vi "RX TX Open (N Channel).vi"(0 "resources":T15[](array[typedef]), 1 "option string":string, 3 "direction":T12, 9 "session in":T1[](array[typedef]), 11 "error in":errorcluster, 12 "force download":bool) -> (4 "tx baseband session out":T2[](array[typedef]), 6 "rx baseband session out":T10[](array[typedef]), 10 "session out":T1[](array[typedef]), 15 "error out":errorcluster)   [LabVIEW 2019]
uses:
  TypeDefs/Resources.ctl
  <vilib>/userDefined/High Color/nirio_resource_hc.ctl
  TypeDefs/Tx Baseband Session.ctl
  <instrlib>/niMmWave/ni3610 and ni3630/controls/public/Main Settings.ctl
  <vilib>/Instr/_visa.llb/VISA Register Access Address Space.ctl
  <instrlib>/niMmWave/ni3610 and ni3630/controls/public/Register Adresses.ctl
  <instrlib>/niMmWave/ni3610 and ni3630/controls/public/Base Card Type.ctl
  <instrlib>/niMmWave/ni3610 and ni3630/controls/private/IQ Card Revision.ctl
  <instrlib>/niMmWave/ni3610 and ni3630/controls/public/Board Capability.ctl
  TypeDefs/Blank FPGA Reference.ctl
  TypeDefs/Rx Baseband Session.ctl
  TypeDefs/Direction.ctl
  TypeDefs/Session.ctl
  <instrlib>/niMmWave/ni3620/Config/v1/Host/Public/High-Level/niMmWave Session.ctl
  <instrlib>/_niInstr/Register Bus/v0/Host/Public/Register Bus Session.ctl
  <instrlib>/_niInstr/Register Bus/v0/Host/Private/Session Data.ctl
  <instrlib>/niMmWave/ni3620/Config/v1/Host/Public/Typedefs/Board Information.ctl
  <instrlib>/niMmWave/ni3620/Config/v1/Host/Public/Typedefs/Hardware Revision.ctl
  <instrlib>/niMmWave/ni3620/Config/v1/Host/Public/Typedefs/Gain Mapping.ctl
  <instrlib>/niMmWave/ni3620/Config/v1/Host/Public/Typedefs/Correction Data.ctl
  <instrlib>/niMmWave/ni3620/Config/v1/Host/Public/Typedefs/Opera Characterization.ctl
  <instrlib>/niMmWave/ni3620/Config/v1/Host/Public/Corrections/Typedefs/Opera Characterization Main Header.ctl
  <instrlib>/niMmWave/ni3620/Config/v1/Host/Public/Corrections/Typedefs/Opera IF Board Information.ctl
  <instrlib>/niMmWave/ni3620/Config/v1/Host/Public/Corrections/Typedefs/Opera Characterization Instance Header.ctl
  <instrlib>/niMmWave/ni3620/Config/v1/Host/Public/Corrections/Typedefs/Opera Characterization Device Data Header.ctl
  <instrlib>/niMmWave/ni3620/Config/v1/Host/Public/Corrections/Typedefs/Opera LO Characterization Data Header.ctl
  <instrlib>/niMmWave/ni3620/Config/v1/Host/Public/Corrections/Typedefs/Opera IF Board Characterization Data Header.ctl
  <instrlib>/niMmWave/ni3620/Config/v1/Host/Public/Corrections/Typedefs/Opera Characterization Device Data.ctl
  <instrlib>/niMmWave/ni3620/Config/v1/Host/Public/Corrections/Typedefs/Opera LO2 Board Characterization Data.ctl
  <instrlib>/niMmWave/ni3620/Config/v1/Host/Public/Corrections/Typedefs/Opera LO Characterization Data.ctl
  <instrlib>/niMmWave/ni3620/Config/v1/Host/Public/Corrections/Typedefs/Opera IF Board Characterization Data.ctl
  <instrlib>/niMmWave/ni3620/Config/v1/Host/Public/Corrections/Typedefs/Opera IQ Impairment Data.ctl
  <instrlib>/niMmWave/ni3620/Config/v1/Host/Public/Typedefs/mmWave Adapter Session Data.ctl
  <instrlib>/niMmWave/ni3620/Config/v1/Host/Public/Typedefs/mmWave Adapter Data.ctl
  <instrlib>/niMmWave/ni3620/Config/v1/Host/Public/Typedefs/mmWave Adapter 2.ctl
  <instrlib>/niMmWave/ni3620/Config/v1/Shared/Typedefs/Subsystem ID.ctl
  <instrlib>/niMmWave/ni3620/Config/v1/Host/Public/Typedefs/mmWave Adapter Channel Information.ctl
  <instrlib>/niMmWave/ni3620/Config/v1/Host/Public/Typedefs/Temperature Coefficients.ctl
  <instrlib>/niMmWave/ni3620/Config/v1/Host/Public/Typedefs/mmWave Characterization.ctl
  <instrlib>/niMmWave/ni3620/Config/v1/Host/Public/Corrections/Typedefs/mmWave Characterization Main Header.ctl
  <instrlib>/niMmWave/ni3620/Config/v1/Host/Public/Corrections/Typedefs/mmWave Characterization Instance Header.ctl
  <instrlib>/niMmWave/ni3620/Config/v1/Host/Public/Typedefs/Session Cache.ctl
  <instrlib>/niMmWave/ni3620/Config/v1/Host/Public/Typedefs/LO2 settings cache.ctl
  <instrlib>/niMmWave/ni3620/Config/v1/Host/Public/Typedefs/LO2 source.ctl
  <instrlib>/niMmWave/ni3620/Config/v1/Host/Public/Typedefs/Desired and Coerced.ctl
  <instrlib>/niMmWave/ni3620/Config/v1/Host/Public/Typedefs/Export cache.ctl
  <instrlib>/niMmWave/ni3620/Config/v1/Host/Public/Typedefs/Path cache.ctl
  <instrlib>/niMmWave/ni3620/Config/v1/Host/Public/Typedefs/Daughterboard Type.ctl
  <instrlib>/niMmWave/ni3620/Config/v1/Host/Public/Typedefs/LO1 settings cache.ctl
  <instrlib>/niMmWave/ni3620/Config/v1/Host/Public/Typedefs/LO1 Source.ctl
  <instrlib>/niMmWave/ni3620/Config/v1/Host/Public/Typedefs/mmWave export cache.ctl
  <instrlib>/niMmWave/ni3620/Config/v1/Host/Private/Board/LO2/LO2 Board Configuration Cache.ctl
  <instrlib>/niMmWave/ni3620/Config/v1/Host/Public/Typedefs/reference clock routing settings.ctl
  <instrlib>/niMmWave/ni3620/Config/v1/Host/Public/Typedefs/LO2 routing settings.ctl
  <instrlib>/niMmWave/ni3620/Config/v1/Host/Private/Board/LO1/LO1 Board Configuration Cache.ctl
  <instrlib>/niMmWave/ni3620/Config/v1/Host/Public/Typedefs/LO1 source settings.ctl
  <instrlib>/niMmWave/ni3620/Config/v1/Host/Public/Typedefs/LO1 export settings.ctl
  <instrlib>/niMmWave/ni3620/Config/v1/Host/Public/Typedefs/LO1 mmWave settings.ctl
  TypeDefs/Hardware Configuration.ctl
  TypeDefs/Gain Ranging.ctl
  TypeDefs/PXI Trigger Bus Info.ctl
  <instrlib>/niMmWave/ni3610 and ni3630/controls/public/Converter Path Selector.ctl
  TypeDefs/RX FPGA Reference.ctl
  Sync/Tclk Parameters.ctl
  TypeDefs/TX FPGA Reference.ctl
  <vilib>/FPGAPlugInAG/PXIe-7902R/niLvFpga_Open_PXIe-7902R.vi
  <vilib>/rvi/interface/common/dynamic/niFpgaDynamicAddResources.vi
  <vilib>/FPGAPlugInAG/Dynamic/niLvFpga_Download_Dynamic.vi
  <vilib>/FPGAPlugInAG/Dynamic/niLvFpga_Run_Dynamic.vi
  <vilib>/Utility/error.llb/Error Cluster From Error Code.vi
  <vilib>/rvi/errors/niLvFpgaAdjustHostInterfaceError.vi
  <vilib>/rvi/interface/nirviOpenFPGA/nirviOpenFPGA.xnode
  FPGA Bitfiles/RX_FPGA_driver_DRAM_v1_2.lvbitx
  <vilib>/rvi/interface/nirviMethod/nirviMethod.xnode
  FPGA Bitfiles/TX_FPGA_driver_DRAM_v1_2_1.lvbitx
  <vilib>/rvi/interface/nirviReadWriteControl/nirviReadWriteControl.xnode
  <instrlib>/niMmWave/ni3610 and ni3630/ni3610_and_ni3630_Driver_Lib.lvlib
  <vilib>/rvi/interface/Simulation/niFpgaSimulationCallBeginRW.vi
  NiFpgaLv.dll
  <instrlib>/niMmWave/ni3620/Config/v1/Host/niMmWave Config v1 Host.lvlib
  <instrlib>/niMmWave/ni3620/Config/v1/Shared/niMmWave Config v1 Shared.lvlib
  <instrlib>/_niInstr/Register Bus/v0/Host/niInstr Register Bus v0 Host.lvlib
panel:
  out "measured skew (samples)":dbl[](array[numeric])
  in  "bypass internal DAC PLL":bool
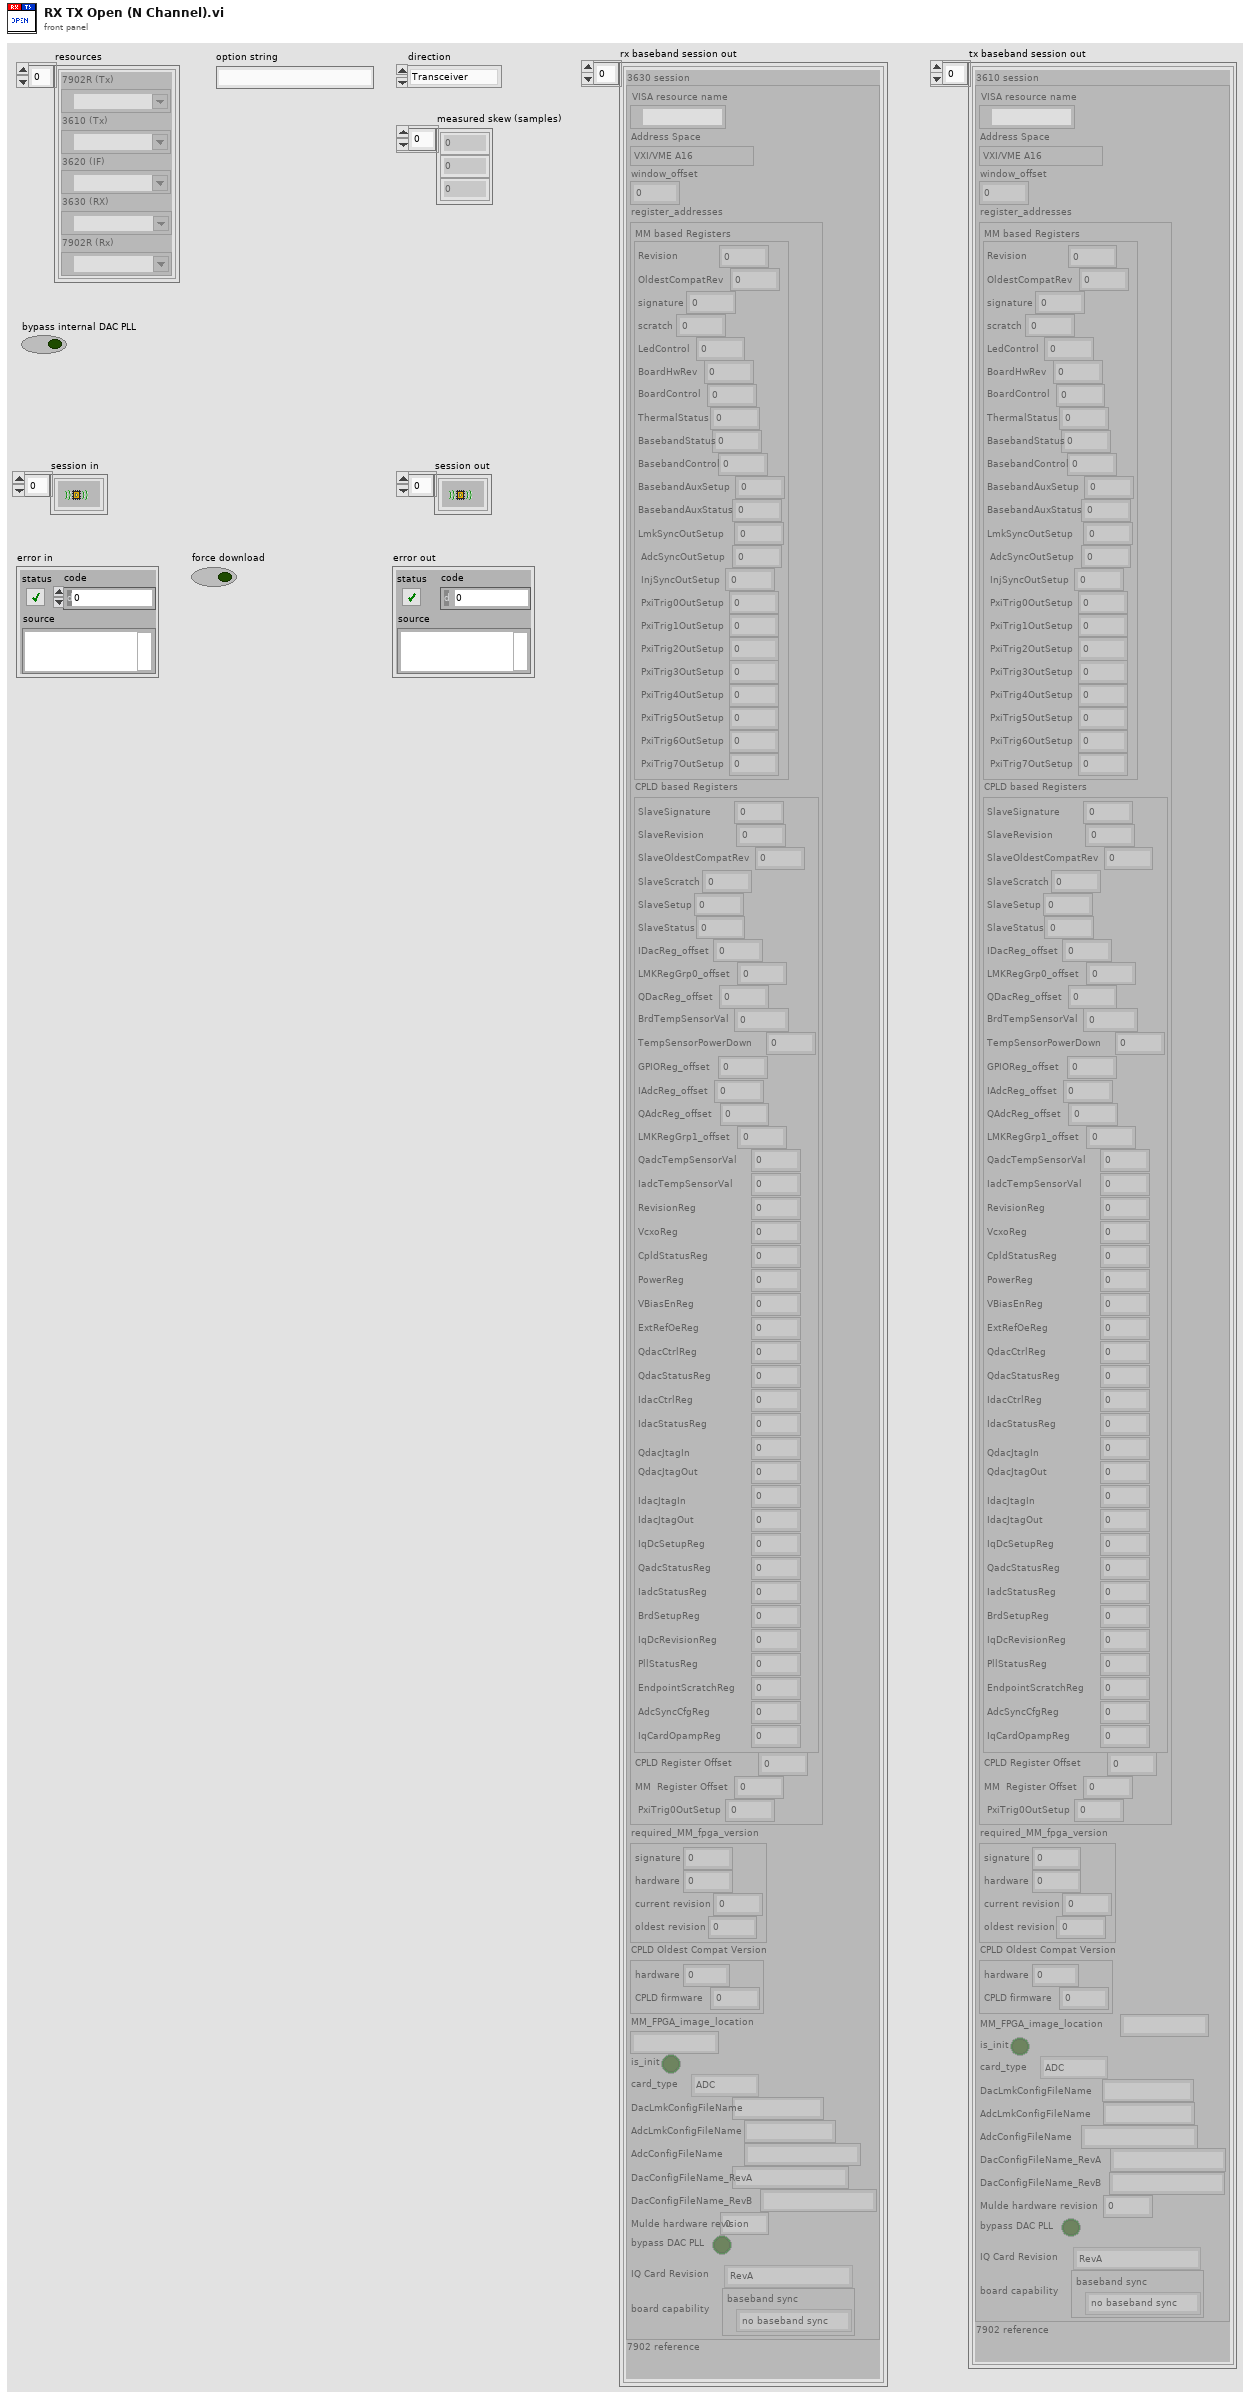
[diagram p1: front panel]
types:
  T1 = typedef "Session.ctl" = cluster{"3620 session":refnum<queue>, "tx baseband session":T2, "rx baseband session":T10, "tx gain (dB)":dbl, "rx gain (dB)":dbl, "hardware configuration":T11, "gain ranging":T13[], "pxi trigger bus information":T14}
  T2 = typedef "Tx Baseband Session.ctl" = cluster{"3610 session":T3, "7902 reference":T9}
  T3 = typedef "ni3610_and_ni3630_Driver_Lib.lvlib/Main Settings.ctl" = cluster{"VISA resource name":refnum<visa-resource-name>, "Address Space":T4, "window_offset":u32, "register_addresses":T5, "required_MM_fpga_version":cluster{"signature":u32, "hardware":u32, "current revision":u32, "oldest revision":u32}, "CPLD Oldest Compat Version ":cluster{"hardware":u32, "CPLD firmware":u32}, "MM_FPGA_image_location":string, "is_init":bool, "card_type":T6, "DacLmkConfigFileName":string, "AdcLmkConfigFileName":string, "AdcConfigFileName":string, "DacConfigFileName_RevA":string, "DacConfigFileName_RevB":string, "Mulde hardware revision":u8, "bypass DAC PLL\n":bool, "IQ Card Revision":T7, "board capability":T8}
  T4 = typedef "VISA Register Access Address Space.ctl" = u16
  T5 = typedef "ni3610_and_ni3630_Driver_Lib.lvlib/Register Adresses.ctl" = cluster{"MM based Registers":cluster{"Revision":u32, "OldestCompatRev":u32, "signature":u32, "scratch":u32, "LedControl":u32, "BoardHwRev":u32, "BoardControl":u32, "ThermalStatus":u32, "BasebandStatus":u32, "BasebandControl":u32, "BasebandAuxSetup":u32, "BasebandAuxStatus":u32, "LmkSyncOutSetup":u32, " AdcSyncOutSetup":u32, " InjSyncOutSetup":u32, " PxiTrig0OutSetup":u32, " PxiTrig1OutSetup":u32, " PxiTrig2OutSetup":u32, " PxiTrig3OutSetup":u32, " PxiTrig4OutSetup":u32, " PxiTrig5OutSetup":u32, " PxiTrig6OutSetup":u32, " PxiTrig7OutSetup":u32}, "CPLD based Registers":cluster{"SlaveSignature":u32, "SlaveRevision":u32, "SlaveOldestCompatRev":u32, "SlaveScratch":u32, "SlaveSetup":u32, "SlaveStatus":u32, "IDacReg_offset":u32, "LMKRegGrp0_offset":u32, "QDacReg_offset":u32, "BrdTempSensorVal":u32, "TempSensorPowerDown":u32, "GPIOReg_offset":u32, "IAdcReg_offset":u32, "QAdcReg_offset":u32, "LMKRegGrp1_offset":u32, "QadcTempSensorVal":u32, "IadcTempSensorVal":u32, "RevisionReg":u32, "VcxoReg":u32, "CpldStatusReg":u32, "PowerReg":u32, "VBiasEnReg":u32, "ExtRefOeReg":u32, "QdacCtrlReg":u32, "QdacStatusReg":u32, "IdacCtrlReg":u32, "IdacStatusReg":u32, "QdacJtagIn":u32, "QdacJtagOut":u32, "IdacJtagIn":u32, "IdacJtagOut":u32, "IqDcSetupReg":u32, "QadcStatusReg":u32, "IadcStatusReg":u32, "BrdSetupReg":u32, "IqDcRevisionReg":u32, "PllStatusReg":u32, "EndpointScratchReg":u32, "AdcSyncCfgReg":u32, "IqCardOpampReg":u32}, "CPLD Register Offset":u32, "MM  Register Offset":u32, " PxiTrig0OutSetup":u32}
  T6 = typedef "ni3610_and_ni3630_Driver_Lib.lvlib/Base Card Type.ctl" = enum16{"unspecified", "ADC", "DAC"}
  T7 = typedef "ni3610_and_ni3630_Driver_Lib.lvlib/IQ Card Revision.ctl" = enum16{"RevA", "RevB", "RevC", "RevD"}
  T8 = typedef "ni3610_and_ni3630_Driver_Lib.lvlib/Board Capability.ctl" = cluster{"baseband sync":enum16{"no baseband sync", "baseband sync"}}
  T9 = typedef "Blank FPGA Reference.ctl" = refnum<k20>
  T10 = typedef "Rx Baseband Session.ctl" = cluster{"3630 session":T3, "7902 reference":T9}
  T11 = typedef "Hardware Configuration.ctl" = cluster{"direction":T12, "baseband only":bool}
  T12 = typedef "Direction.ctl" = enum16{"Transceiver", "Receiver", "Transmitter"}
  T13 = typedef "Gain Ranging.ctl" = cluster{"gain ranging active scope":string, "gain ranging stream session":refnum<k20>}
  T14 = typedef "PXI Trigger Bus Info.ctl" = cluster{"chassis resource name":refnum<visa-resource-name>, "7902R (TX)":i16, "3610 (TX)":i16, "3620 (IF)":i16, "3630 (RX)":i16, "7902R (RX)":i16}
  T15 = typedef "Resources.ctl" = cluster{"7902R (Tx)":T16, "3610 (Tx)":refnum<visa-resource-name>, "3620 (IF)":T16, "3630 (RX)":refnum<visa-resource-name>, "7902R (Rx)":T16}
  T16 = typedef "nirio_resource_hc.ctl" = tag
  T17 = typedef "Tclk Parameters.ctl" = cluster{"tclk divider":u16, "fpga data clock (Hz)":dbl, "sample rate (Hz)":dbl}
  T18 = typedef "RX FPGA Reference.ctl" = refnum<k20>
  T19 = typedef "TX FPGA Reference.ctl" = refnum<k20>
  T20 = typedef "Constants.ctl" = cluster{"data clock rate (Hz)":dbl, "sample rate (Hz)":dbl, "sample rate selector string":string, "default tx bitfile path":path, "default rx bitfile path":path, "default proc bitfile path":path}
  T21 = typedef "Baseband Resources.ctl" = cluster{"chevelle resource":T16, "mulde resource":refnum<visa-resource-name>}
  T22 = enum16{"TClk Trigger", "TClk Measure", "ADC Sync Injection", "Tx JESD Sync", "Rx JESD Sync", "Tx ADC Sync Injection", "Tx Master10k_Reset"}[]
  T23 = typedef "ni3610_and_ni3630_Driver_Lib.lvlib/Converter Path Selector.ctl" = enum16{"I-path device", "Q-path device"}
  T24 = typedef "ni3610_and_ni3630_Driver_Lib.lvlib/Baseband IQ Characterization Device Data.ctl" = cluster{"Checksum":u32, "Channel Delay":dbl, "Imbalance":cluster{"Gain Imbalance":dbl, "Phase Imbalance":dbl}, "DC Offset":cluster{"I DC Offset":dbl, "Q DC Offset":dbl}}
  T25 = cluster{"reset":bool, "gtx enable":bool, "jesd enable":bool, "sw sync":bool, "gtx post cursor":fxp<+,5,5>, "gtx pre cursor":fxp<+,5,5>, "gtx diff control":fxp<+,4,4>, "clock enable":bool, "lmfc delay":fxp<+,5,5>, "sysref enable":bool, "sync enable":bool, "trig7 listen":bool, "trig7 invert":bool, "clear data in error":bool}
diagram:
  n1 = case shown="No Error" "error in" {
    selector: "error in" -> [w47 w461]
    tunnel: "option string" -> [w51 _]
    tunnel: "resources" -> [w45 _]
    tunnel: [w49 _] -> w8
    tunnel: [w32 _] -> w6
    tunnel: [w33 _] -> w7
    tunnel: [w34 w461] -> w9
    tunnel: "force download" -> [w50 _]
    tunnel: "bypass internal DAC PLL" -> [w48 _]
    tunnel: "direction" -> [w15 _]
    tunnel: "session in" -> [w20 _]
    tunnel: [w20 _] -> w1
    frame No Error {
      n2 = call "Get Constants.vi"() -> ("constants"=w53:T20)  [unwired: 15 in]
      n3 = call "Get Rx Tx resources.vi"("resources"=w45, "direction"=w15, "error in (no error)"=w47) -> ("RX Resources"=w36:T21[], "TX Resources"=w35:T21[], "error out"=w46:errorcluster)  [unwired: 10 in]
      n4 = Unbundle By Name(w53) -> ("sample rate (Hz)"=w39:dbl)  [unwired: 1 out]
      n5 = case shown="\"Transceiver\", \"Receiver\"" w15 {
        tunnel: [w77 w86] -> w52
        tunnel: w51 -> [_ w85]
        tunnel: w46 -> [w77 w84]
        tunnel: [w78 w83] -> w28
        tunnel: w36 -> [_ w80]
        tunnel: [w76 w82] -> w18
        tunnel: w50 -> [_ w81]
        frame "Transmitter" {
          n6 = Initialize Array(T3 {"VISA resource name"=refnum, "Address Space"=0, "window_offset"=0, "register_addresses"={"MM based Registers"={"Revision"=0, "OldestCompatRev"=0, "signature"=0, "scratch"=0, "LedControl"=0, "BoardHwRev"=0, "BoardControl"=0, "ThermalStatus"=0, "BasebandStatus"=0, "BasebandControl"=0, "BasebandAuxSetup"=0, "BasebandAuxStatus"=0, "LmkSyncOutSetup"=0, " AdcSyncOutSetup"=0, " InjSyncOutSetup"=0, " PxiTrig0OutSetup"=0, " PxiTrig1OutSetup"=0, " PxiTrig2OutSetup"=0, " PxiTrig3OutSetup"=0, " PxiTrig4OutSetup"=0, " PxiTrig5OutSetup"=0, " PxiTrig6OutSetup"=0, " PxiTrig7OutSetup"=0}, "CPLD based Registers"={"SlaveSignature"=0, "SlaveRevision"=0, "SlaveOldestCompatRev"=0, "SlaveScratch"=0, "SlaveSetup"=0, "SlaveStatus"=0, "IDacReg_offset"=0, "LMKRegGrp0_offset"=0, "QDacReg_offset"=0, "BrdTempSensorVal"=0, "TempSensorPowerDown"=0, "GPIOReg_offset"=0, "IAdcReg_offset"=0, "QAdcReg_offset"=0, "LMKRegGrp1_offset"=0, "QadcTempSensorVal"=0, "IadcTempSensorVal"=0, "RevisionReg"=0, "VcxoReg"=0, "CpldStatusReg"=0, "PowerReg"=0, "VBiasEnReg"=0, "ExtRefOeReg"=0, "QdacCtrlReg"=0, "QdacStatusReg"=0, "IdacCtrlReg"=0, "IdacStatusReg"=0, "QdacJtagIn"=0, "QdacJtagOut"=0, "IdacJtagIn"=0, "IdacJtagOut"=0, "IqDcSetupReg"=0, "QadcStatusReg"=0, "IadcStatusReg"=0, "BrdSetupReg"=0, "IqDcRevisionReg"=0, "PllStatusReg"=0, "EndpointScratchReg"=0, "AdcSyncCfgReg"=0, "IqCardOpampReg"=0}, "CPLD Register Offset"=0, "MM  Register Offset"=0, " PxiTrig0OutSetup"=0}, "required_MM_fpga_version"={"signature"=0, "hardware"=0, "current revision"=0, "oldest revision"=0}, "CPLD Oldest Compat Version "={"hardware"=0, "CPLD firmware"=0}, "MM_FPGA_image_location"="", "is_init"=FALSE, "card_type"=enum."ADC", "DacLmkConfigFileName"="", "AdcLmkConfigFileName"="", "AdcConfigFileName"="", "DacConfigFileName_RevA"="", "DacConfigFileName_RevB"="", "Mulde hardware revision"=0, "bypass DAC PLL\n"=FALSE, "IQ Card Revision"=enum."RevA", "board capability"={"baseband sync"=enum."no baseband sync"}}) -> (w78:T3[])  [unwired: 1 in]
          n7 = Initialize Array(refnum<k20> refnum) -> (w76:refnum<k20>[])  [unwired: 1 in]
        }
        frame "Transceiver", "Receiver" {
          n8 = for {
            tunnel: w80 -> [w100] mode=indexing
            shift-right: [w98] -> w86
            shift-left: w84 -> [w91]
            tunnel: w85 -> [w97]
            tunnel: w81 -> [w95]
            tunnel: [w94] -> w83 mode=indexing
            tunnel: [w93] -> w82 mode=indexing
            # "RX FPGA:\nRX_FPGA_driver_DRAM_v1_2.lvbitx"
            # "RX\nDownload bitfile and power up ADC (3630)"
            n9 = Unbundle By Name(w100) -> ("mulde resource"=w96:refnum<visa-resource-name>, "chevelle resource"=w92:T16)
            n10 = xnode "Open FPGA VI Reference"("error in"=w91, "resource name"=w92) -> ("FPGA VI Reference Out"=w87:refnum<k20>, "error out"=w90:errorcluster)
            n11 = Dynamic FPGA Interface Cast(Session In=T9 refnum, Type=w87) -> (Session Out=w89:T9)
            n12 = case shown="True" w95 {
              tunnel: w89 -> [w102 w108]
              tunnel: [w101 w106] -> w99
              tunnel: w90 -> [w101 w105]
              tunnel: [w102 w103] -> w93
              frame False {
              }
              frame True {
                n13 = xnode "Invoke Method"("FPGA VI Reference In"=w108, "error in"=w105) -> ("FPGA VI Reference Out"=w107:T9, "error out"=w104:errorcluster)
                n14 = xnode "Invoke Method"("FPGA VI Reference In"=w107, "error in"=w104) -> ("FPGA VI Reference Out"=w103:T9, "error out"=w106:errorcluster)  [unwired: 1 in]
              }
            }
            n15 = case shown="No Error" w99 {
              selector: w99 -> [w110 w124]
              tunnel: w96 -> [w109 _]
              tunnel: [w112 w124] -> w98
              tunnel: w97 -> [w113 _]
              tunnel: [w111 T3 {"VISA resource name"=refnum, "Address Space"=0, "window_offset"=0, "register_addresses"={"MM based Registers"={"Revision"=0, "OldestCompatRev"=0, "signature"=0, "scratch"=0, "LedControl"=0, "BoardHwRev"=0, "BoardControl"=0, "ThermalStatus"=0, "BasebandStatus"=0, "BasebandControl"=0, "BasebandAuxSetup"=0, "BasebandAuxStatus"=0, "LmkSyncOutSetup"=0, " AdcSyncOutSetup"=0, " InjSyncOutSetup"=0, " PxiTrig0OutSetup"=0, " PxiTrig1OutSetup"=0, " PxiTrig2OutSetup"=0, " PxiTrig3OutSetup"=0, " PxiTrig4OutSetup"=0, " PxiTrig5OutSetup"=0, " PxiTrig6OutSetup"=0, " PxiTrig7OutSetup"=0}, "CPLD based Registers"={"SlaveSignature"=0, "SlaveRevision"=0, "SlaveOldestCompatRev"=0, "SlaveScratch"=0, "SlaveSetup"=0, "SlaveStatus"=0, "IDacReg_offset"=0, "LMKRegGrp0_offset"=0, "QDacReg_offset"=0, "BrdTempSensorVal"=0, "TempSensorPowerDown"=0, "GPIOReg_offset"=0, "IAdcReg_offset"=0, "QAdcReg_offset"=0, "LMKRegGrp1_offset"=0, "QadcTempSensorVal"=0, "IadcTempSensorVal"=0, "RevisionReg"=0, "VcxoReg"=0, "CpldStatusReg"=0, "PowerReg"=0, "VBiasEnReg"=0, "ExtRefOeReg"=0, "QdacCtrlReg"=0, "QdacStatusReg"=0, "IdacCtrlReg"=0, "IdacStatusReg"=0, "QdacJtagIn"=0, "QdacJtagOut"=0, "IdacJtagIn"=0, "IdacJtagOut"=0, "IqDcSetupReg"=0, "QadcStatusReg"=0, "IadcStatusReg"=0, "BrdSetupReg"=0, "IqDcRevisionReg"=0, "PllStatusReg"=0, "EndpointScratchReg"=0, "AdcSyncCfgReg"=0, "IqCardOpampReg"=0}, "CPLD Register Offset"=0, "MM  Register Offset"=0, " PxiTrig0OutSetup"=0}, "required_MM_fpga_version"={"signature"=0, "hardware"=0, "current revision"=0, "oldest revision"=0}, "CPLD Oldest Compat Version "={"hardware"=0, "CPLD firmware"=0}, "MM_FPGA_image_location"="", "is_init"=FALSE, "card_type"=enum."ADC", "DacLmkConfigFileName"="", "AdcLmkConfigFileName"="", "AdcConfigFileName"="", "DacConfigFileName_RevA"="", "DacConfigFileName_RevB"="", "Mulde hardware revision"=0, "bypass DAC PLL\n"=FALSE, "IQ Card Revision"=enum."RevA", "board capability"={"baseband sync"=enum."no baseband sync"}}] -> w94
              frame No Error {
                (unwired) T10 {"3630 session"={"VISA resource name"=refnum, "Address Space"=1, "window_offset"=0, "register_addresses"={"MM based Registers"={"Revision"=0, "OldestCompatRev"=0, "signature"=0, "scratch"=0, "LedControl"=0, "BoardHwRev"=0, "BoardControl"=0, "ThermalStatus"=0, "BasebandStatus"=0, "BasebandControl"=0, "BasebandAuxSetup"=0, "BasebandAuxStatus"=0, "LmkSyncOutSetup"=0, " AdcSyncOutSetup"=0, " InjSyncOutSetup"=0, " PxiTrig0OutSetup"=0, " PxiTrig1OutSetup"=0, " PxiTrig2OutSetup"=0, " PxiTrig3OutSetup"=0, " PxiTrig4OutSetup"=0, " PxiTrig5OutSetup"=0, " PxiTrig6OutSetup"=0, " PxiTrig7OutSetup"=0}, "CPLD based Registers"={"SlaveSignature"=0, "SlaveRevision"=0, "SlaveOldestCompatRev"=0, "SlaveScratch"=0, "SlaveSetup"=0, "SlaveStatus"=0, "IDacReg_offset"=0, "LMKRegGrp0_offset"=0, "QDacReg_offset"=0, "BrdTempSensorVal"=0, "TempSensorPowerDown"=0, "GPIOReg_offset"=0, "IAdcReg_offset"=0, "QAdcReg_offset"=0, "LMKRegGrp1_offset"=0, "QadcTempSensorVal"=0, "IadcTempSensorVal"=0, "RevisionReg"=0, "VcxoReg"=0, "CpldStatusReg"=0, "PowerReg"=0, "VBiasEnReg"=0, "ExtRefOeReg"=0, "QdacCtrlReg"=0, "QdacStatusReg"=0, "IdacCtrlReg"=0, "IdacStatusReg"=0, "QdacJtagIn"=0, "QdacJtagOut"=0, "IdacJtagIn"=0, "IdacJtagOut"=0, "IqDcSetupReg"=0, "QadcStatusReg"=0, "IadcStatusReg"=0, "BrdSetupReg"=0, "IqDcRevisionReg"=0, "PllStatusReg"=0, "EndpointScratchReg"=0, "AdcSyncCfgReg"=0, "IqCardOpampReg"=0}, "CPLD Register Offset"=0, "MM  Register Offset"=0, " PxiTrig0OutSetup"=0}, "required_MM_fpga_version"={"signature"=0, "hardware"=0, "current revision"=0, "oldest revision"=0}, "CPLD Oldest Compat Version "={"hardware"=0, "CPLD firmware"=0}, "MM_FPGA_image_location"="", "is_init"=FALSE, "card_type"=enum."ADC", "DacLmkConfigFileName"="", "AdcLmkConfigFileName"="", "AdcConfigFileName"="", "DacConfigFileName_RevA"="", "DacConfigFileName_RevB"="", "Mulde hardware revision"=0, "bypass DAC PLL\n"=FALSE, "IQ Card Revision"=enum."RevA", "board capability"={"baseband sync"=enum."no baseband sync"}}, "7902 reference"=refnum}
                n16 = case shown="No Error" w110 {
                  selector: w110 -> [w119 w122]
                  tunnel: [w115 w122] -> w112
                  tunnel: w109 -> [w120 _]
                  tunnel: [w116 T3 {"VISA resource name"=refnum, "Address Space"=0, "window_offset"=0, "register_addresses"={"MM based Registers"={"Revision"=0, "OldestCompatRev"=0, "signature"=0, "scratch"=0, "LedControl"=0, "BoardHwRev"=0, "BoardControl"=0, "ThermalStatus"=0, "BasebandStatus"=0, "BasebandControl"=0, "BasebandAuxSetup"=0, "BasebandAuxStatus"=0, "LmkSyncOutSetup"=0, " AdcSyncOutSetup"=0, " InjSyncOutSetup"=0, " PxiTrig0OutSetup"=0, " PxiTrig1OutSetup"=0, " PxiTrig2OutSetup"=0, " PxiTrig3OutSetup"=0, " PxiTrig4OutSetup"=0, " PxiTrig5OutSetup"=0, " PxiTrig6OutSetup"=0, " PxiTrig7OutSetup"=0}, "CPLD based Registers"={"SlaveSignature"=0, "SlaveRevision"=0, "SlaveOldestCompatRev"=0, "SlaveScratch"=0, "SlaveSetup"=0, "SlaveStatus"=0, "IDacReg_offset"=0, "LMKRegGrp0_offset"=0, "QDacReg_offset"=0, "BrdTempSensorVal"=0, "TempSensorPowerDown"=0, "GPIOReg_offset"=0, "IAdcReg_offset"=0, "QAdcReg_offset"=0, "LMKRegGrp1_offset"=0, "QadcTempSensorVal"=0, "IadcTempSensorVal"=0, "RevisionReg"=0, "VcxoReg"=0, "CpldStatusReg"=0, "PowerReg"=0, "VBiasEnReg"=0, "ExtRefOeReg"=0, "QdacCtrlReg"=0, "QdacStatusReg"=0, "IdacCtrlReg"=0, "IdacStatusReg"=0, "QdacJtagIn"=0, "QdacJtagOut"=0, "IdacJtagIn"=0, "IdacJtagOut"=0, "IqDcSetupReg"=0, "QadcStatusReg"=0, "IadcStatusReg"=0, "BrdSetupReg"=0, "IqDcRevisionReg"=0, "PllStatusReg"=0, "EndpointScratchReg"=0, "AdcSyncCfgReg"=0, "IqCardOpampReg"=0}, "CPLD Register Offset"=0, "MM  Register Offset"=0, " PxiTrig0OutSetup"=0}, "required_MM_fpga_version"={"signature"=0, "hardware"=0, "current revision"=0, "oldest revision"=0}, "CPLD Oldest Compat Version "={"hardware"=0, "CPLD firmware"=0}, "MM_FPGA_image_location"="", "is_init"=FALSE, "card_type"=enum."ADC", "DacLmkConfigFileName"="", "AdcLmkConfigFileName"="", "AdcConfigFileName"="", "DacConfigFileName_RevA"="", "DacConfigFileName_RevB"="", "Mulde hardware revision"=0, "bypass DAC PLL\n"=FALSE, "IQ Card Revision"=enum."RevA", "board capability"={"baseband sync"=enum."no baseband sync"}}] -> w111
                  tunnel: Base_Card_Type."ADC" -> [w118 _]
                  tunnel: w113 -> [w117 _]
                  frame No Error {
                    # "Combine Initialization Routines"
                    n17 = call <instrlib>:"Board Initialize.vi"("option string"=w117, "error in"=w119, "Base Card Type"=w118, "VISA resource name"=w120) -> ("error out"=w115:errorcluster, "Board Settings out"=w116:T3)  [unwired: 6 in]
                  }
                  frame Error {
                  }
                }
              }
              frame Error {
              }
            }
          }
        }
      }
      n18 = case shown="\"Transceiver\", \"Transmitter\"" w15 {
        tunnel: w52 -> [w127 w136]
        tunnel: w51 -> [_ w135]
        tunnel: [w127 w134] -> w27
        tunnel: [w128 w133] -> w21
        tunnel: w35 -> [_ w132]
        tunnel: [w126 w131] -> w19
        tunnel: w50 -> [_ w130]
        frame "Receiver" {
          n19 = Initialize Array(T3 {"VISA resource name"=refnum, "Address Space"=0, "window_offset"=0, "register_addresses"={"MM based Registers"={"Revision"=0, "OldestCompatRev"=0, "signature"=0, "scratch"=0, "LedControl"=0, "BoardHwRev"=0, "BoardControl"=0, "ThermalStatus"=0, "BasebandStatus"=0, "BasebandControl"=0, "BasebandAuxSetup"=0, "BasebandAuxStatus"=0, "LmkSyncOutSetup"=0, " AdcSyncOutSetup"=0, " InjSyncOutSetup"=0, " PxiTrig0OutSetup"=0, " PxiTrig1OutSetup"=0, " PxiTrig2OutSetup"=0, " PxiTrig3OutSetup"=0, " PxiTrig4OutSetup"=0, " PxiTrig5OutSetup"=0, " PxiTrig6OutSetup"=0, " PxiTrig7OutSetup"=0}, "CPLD based Registers"={"SlaveSignature"=0, "SlaveRevision"=0, "SlaveOldestCompatRev"=0, "SlaveScratch"=0, "SlaveSetup"=0, "SlaveStatus"=0, "IDacReg_offset"=0, "LMKRegGrp0_offset"=0, "QDacReg_offset"=0, "BrdTempSensorVal"=0, "TempSensorPowerDown"=0, "GPIOReg_offset"=0, "IAdcReg_offset"=0, "QAdcReg_offset"=0, "LMKRegGrp1_offset"=0, "QadcTempSensorVal"=0, "IadcTempSensorVal"=0, "RevisionReg"=0, "VcxoReg"=0, "CpldStatusReg"=0, "PowerReg"=0, "VBiasEnReg"=0, "ExtRefOeReg"=0, "QdacCtrlReg"=0, "QdacStatusReg"=0, "IdacCtrlReg"=0, "IdacStatusReg"=0, "QdacJtagIn"=0, "QdacJtagOut"=0, "IdacJtagIn"=0, "IdacJtagOut"=0, "IqDcSetupReg"=0, "QadcStatusReg"=0, "IadcStatusReg"=0, "BrdSetupReg"=0, "IqDcRevisionReg"=0, "PllStatusReg"=0, "EndpointScratchReg"=0, "AdcSyncCfgReg"=0, "IqCardOpampReg"=0}, "CPLD Register Offset"=0, "MM  Register Offset"=0, " PxiTrig0OutSetup"=0}, "required_MM_fpga_version"={"signature"=0, "hardware"=0, "current revision"=0, "oldest revision"=0}, "CPLD Oldest Compat Version "={"hardware"=0, "CPLD firmware"=0}, "MM_FPGA_image_location"="", "is_init"=FALSE, "card_type"=enum."ADC", "DacLmkConfigFileName"="", "AdcLmkConfigFileName"="", "AdcConfigFileName"="", "DacConfigFileName_RevA"="", "DacConfigFileName_RevB"="", "Mulde hardware revision"=0, "bypass DAC PLL\n"=FALSE, "IQ Card Revision"=enum."RevA", "board capability"={"baseband sync"=enum."no baseband sync"}}) -> (w128:T3[])  [unwired: 1 in]
          n20 = Initialize Array(refnum<k20> refnum) -> (w126:refnum<k20>[])  [unwired: 1 in]
        }
        frame "Transceiver", "Transmitter" {
          n21 = for {
            shift-right: [w149] -> w134
            shift-left: w136 -> [w141]
            tunnel: w135 -> [w146]
            tunnel: w132 -> [w148] mode=indexing
            tunnel: w130 -> [w147]
            tunnel: [w144] -> w133 mode=indexing
            tunnel: [w143] -> w131 mode=indexing
            # "TX FPGA:\nTX_FPGA_driver_DRAM_v1_2_1.lvbitx"
            # "TX\nDownload bitfile and power up DAC (3610)"
            n22 = Unbundle By Name(w148) -> ("mulde resource"=w145:refnum<visa-resource-name>, "chevelle resource"=w142:T16)
            n23 = xnode "Open FPGA VI Reference"("error in"=w141, "resource name"=w142) -> ("FPGA VI Reference Out"=w137:refnum<k20>, "error out"=w140:errorcluster)
            n24 = Dynamic FPGA Interface Cast(Session In=T9 refnum, Type=w137) -> (Session Out=w139:T9)
            n25 = case shown="True" w147 {
              tunnel: w139 -> [w168 w174]
              tunnel: [w167 w172] -> w151
              tunnel: w140 -> [w167 w171]
              tunnel: [w168 w169] -> w150
              frame False {
              }
              frame True {
                n26 = xnode "Invoke Method"("FPGA VI Reference In"=w174, "error in"=w171) -> ("FPGA VI Reference Out"=w173:T9, "error out"=w170:errorcluster)
                n27 = xnode "Invoke Method"("FPGA VI Reference In"=w173, "error in"=w170) -> ("FPGA VI Reference Out"=w169:T9, "error out"=w172:errorcluster)  [unwired: 1 in]
              }
            }
            n28 = case shown="No Error" w151 {
              selector: w151 -> [w163 w166]
              tunnel: w150 -> [w153 w165]
              tunnel: w145 -> [w157 _]
              tunnel: [w154 w166] -> w149
              tunnel: [w162 w165] -> w143
              tunnel: [w155 T3 {"VISA resource name"=refnum, "Address Space"=0, "window_offset"=0, "register_addresses"={"MM based Registers"={"Revision"=0, "OldestCompatRev"=0, "signature"=0, "scratch"=0, "LedControl"=0, "BoardHwRev"=0, "BoardControl"=0, "ThermalStatus"=0, "BasebandStatus"=0, "BasebandControl"=0, "BasebandAuxSetup"=0, "BasebandAuxStatus"=0, "LmkSyncOutSetup"=0, " AdcSyncOutSetup"=0, " InjSyncOutSetup"=0, " PxiTrig0OutSetup"=0, " PxiTrig1OutSetup"=0, " PxiTrig2OutSetup"=0, " PxiTrig3OutSetup"=0, " PxiTrig4OutSetup"=0, " PxiTrig5OutSetup"=0, " PxiTrig6OutSetup"=0, " PxiTrig7OutSetup"=0}, "CPLD based Registers"={"SlaveSignature"=0, "SlaveRevision"=0, "SlaveOldestCompatRev"=0, "SlaveScratch"=0, "SlaveSetup"=0, "SlaveStatus"=0, "IDacReg_offset"=0, "LMKRegGrp0_offset"=0, "QDacReg_offset"=0, "BrdTempSensorVal"=0, "TempSensorPowerDown"=0, "GPIOReg_offset"=0, "IAdcReg_offset"=0, "QAdcReg_offset"=0, "LMKRegGrp1_offset"=0, "QadcTempSensorVal"=0, "IadcTempSensorVal"=0, "RevisionReg"=0, "VcxoReg"=0, "CpldStatusReg"=0, "PowerReg"=0, "VBiasEnReg"=0, "ExtRefOeReg"=0, "QdacCtrlReg"=0, "QdacStatusReg"=0, "IdacCtrlReg"=0, "IdacStatusReg"=0, "QdacJtagIn"=0, "QdacJtagOut"=0, "IdacJtagIn"=0, "IdacJtagOut"=0, "IqDcSetupReg"=0, "QadcStatusReg"=0, "IadcStatusReg"=0, "BrdSetupReg"=0, "IqDcRevisionReg"=0, "PllStatusReg"=0, "EndpointScratchReg"=0, "AdcSyncCfgReg"=0, "IqCardOpampReg"=0}, "CPLD Register Offset"=0, "MM  Register Offset"=0, " PxiTrig0OutSetup"=0}, "required_MM_fpga_version"={"signature"=0, "hardware"=0, "current revision"=0, "oldest revision"=0}, "CPLD Oldest Compat Version "={"hardware"=0, "CPLD firmware"=0}, "MM_FPGA_image_location"="", "is_init"=FALSE, "card_type"=enum."ADC", "DacLmkConfigFileName"="", "AdcLmkConfigFileName"="", "AdcConfigFileName"="", "DacConfigFileName_RevA"="", "DacConfigFileName_RevB"="", "Mulde hardware revision"=0, "bypass DAC PLL\n"=FALSE, "IQ Card Revision"=enum."RevA", "board capability"={"baseband sync"=enum."no baseband sync"}}] -> w144
              tunnel: w146 -> [w158 _]
              frame No Error {
                n29 = call "Configure Chevelle JESD TX.vi"("fpga ref in"=w153, "error in (no error)"=w163) -> ("fpga ref out"=w152:T9, "error out"=w160:errorcluster)  [unwired: 12 in]
                n30 = call "Configure IQ Inversion.vi"("fpga reference in"=w152, "iq inversion"=cluster{"invert I":bool, "invert Q":bool} {"invert I"=FALSE, "invert Q"=FALSE}, "error in"=w160) -> ("fpga reference out"=w162:T9, "error out"=w159:errorcluster)  [unwired: 11 in]
                n31 = call <instrlib>:"Board Initialize.vi"("option string"=w158, "error in"=w159, "Base Card Type"=Base_Card_Type."DAC", "VISA resource name"=w157) -> ("error out"=w154:errorcluster, "Board Settings out"=w155:T3)  [unwired: 6 in]
              }
              frame Error {
              }
            }
          }
        }
      }
      n32 = call "Verify Matching Board Capabilities.vi"("TX Board Settings"=w21, "RX Board Settings"=w28, "error in (no error)"=w27) -> ("RX TX Board Settings"=w25:T3[], "error out"=w26:errorcluster)  [unwired: 11 in]
      n33 = Index Array(array=w25, index=0) -> (element=w23:T3)
      n34 = Unbundle By Name(w23) -> ("board capability.baseband sync"=w22:enum16{"no baseband sync", "baseband sync"})
      n35 = case shown="\"no baseband sync\", Default" w22 {
        tunnel: [w219 w237] -> w29
        tunnel: w15 -> [w218 w233]
        tunnel: w26 -> [w220 w232]
        tunnel: w20 -> [w224 w234]
        frame "no baseband sync", Default {
          w221 = TRUE  # map(T)/unmap(F)
          n36 = for {
            tunnel: w224 -> [w226] mode=indexing
            tunnel: [w225] -> w223 mode=indexing
            n37 = Unbundle By Name(w226) -> ("pxi trigger bus information"=w225:T14)
          }
          n38 = case shown="\"Receiver\"" w218 {
            tunnel: [w227 w228 w229] -> w222
            frame "Transmitter" {
              w227 = T22 [enum."TClk Measure", enum."TClk Trigger", enum."Tx JESD Sync"] items=["TClk Trigger", "TClk Measure", "ADC Sync Injection", "Tx JESD Sync", "Rx JESD Sync", "Tx ADC Sync Injection", "Tx Master10k_Reset"]
            }
            frame "Transceiver" {
              w228 = T22 [enum."TClk Measure", enum."TClk Trigger", enum."ADC Sync Injection", enum."Tx JESD Sync", enum."Rx JESD Sync"] items=["TClk Trigger", "TClk Measure", "ADC Sync Injection", "Tx JESD Sync", "Rx JESD Sync", "Tx ADC Sync Injection", "Tx Master10k_Reset"]
            }
            frame "Receiver" {
              w229 = T22 [enum."TClk Measure", enum."TClk Trigger", enum."ADC Sync Injection", enum."Rx JESD Sync"] items=["TClk Trigger", "TClk Measure", "ADC Sync Injection", "Tx JESD Sync", "Rx JESD Sync", "Tx ADC Sync Injection", "Tx Master10k_Reset"]
            }
          }
          n39 = call "Route Triggers.vi"("pxi trigger bus configuration [channel]"=w223, "route for"=w222, "map(T)/unmap(F)"=w221, "Direction"=w218, "error in"=w220) -> ("error out"=w219:errorcluster)  [unwired: 10 in]
        }
        frame "baseband sync" {
          w235 = TRUE  # map(T)/unmap(F)
          # "Set up PXI_6 and PXI_7 trigger routing for\nDAC moudles (3610) that supports baseband synchronization"
          n40 = case shown="\"Transceiver\"" w233 {
            tunnel: [w240 w241 w242] -> w236
            frame "Transmitter" {
              w240 = T22 [enum."TClk Measure", enum."TClk Trigger", enum."Tx ADC Sync Injection", enum."Tx Master10k_Reset"] items=["TClk Trigger", "TClk Measure", "ADC Sync Injection", "Tx JESD Sync", "Rx JESD Sync", "Tx ADC Sync Injection", "Tx Master10k_Reset"]
            }
            frame "Transceiver" {
              w241 = T22 [enum."TClk Trigger", enum."Rx JESD Sync", enum."Tx ADC Sync Injection", enum."Tx Master10k_Reset"] items=["TClk Trigger", "TClk Measure", "ADC Sync Injection", "Tx JESD Sync", "Rx JESD Sync", "Tx ADC Sync Injection", "Tx Master10k_Reset"]
            }
            frame "Receiver" {
              w242 = T22 [enum."TClk Measure", enum."TClk Trigger", enum."ADC Sync Injection", enum."Rx JESD Sync"] items=["TClk Trigger", "TClk Measure", "ADC Sync Injection", "Tx JESD Sync", "Rx JESD Sync", "Tx ADC Sync Injection", "Tx Master10k_Reset"]
            }
          }
          n41 = for {
            tunnel: w234 -> [w239] mode=indexing
            tunnel: [w238] -> w230 mode=indexing
            n42 = Unbundle By Name(w239) -> ("pxi trigger bus information"=w238:T14)
          }
          n43 = call "Check Multichassis Sync Support.vi"("error in (no error)"=w232, "pxi trigger bus configuration [channel]"=w230) -> ("error out"=w231:errorcluster)  [unwired: 9 in]